vi "SPCReadFile.vi"(8 "Error In":errorcluster, 9 "Save data to ASCII":bool, 11 "SPC File":path) -> (0 "Error Out":errorcluster, 1 "Time Axis Multiplicator":dbl=0.01221522705078125, 2 "Events":u16[](array[numeric]) format="%04x", 3 "SumOfDecays":u32[](graph)=[0, 0, 0, 0, 0, 0, 0, 0, 0, 0, 0, 0, 0, 0, 0, 0, 0, 0, 0, 0, 0, 0, 0, 0, 0, 0, 0, 0, 0, 0, 0, 0, 0, 0, 0, 0, 0, 0, 0, 0, 0, 0, 0, 0, 0, 0, 0, 0, 0, 0, 0, 0, 0, 0, 0, 0, 0, 0, 0, 0, 0, 0, 0, 0, 0, 0, 0, 0, 0, 0, 0, 0, 0, 0, 0, 0, 0, 0, 0, 0, 0, 0, 0, 0, 0, 0, 0, 0, 0, 0, 0, 0, 0, 0, 0, 0, 0, 0, 0, 0, 0, 0, 0, 0, 0, 0, 0, 0, 0, 0, 0, 0, 0, 0, 0, 0, 0, 0, 0, 0, 0, 0, 0, 0, 0, 0, 0, 0, 0, 0, 0, 0, 0, 0, 0, 0, 0, 0, 0, 0, 0, 0, 0, 0, 0, 0, 0, 0, 0, 0, 0, 0, 0, 0, 0, 0, 0, 0, 0, 0, 0, 0, 0, 0, 0, 0, 0, 0, 0, 0, 0, 0, 0, 0, 0, 0, 0, 0, 0, 0, 0, 0, 0, 0, 0, 0, 0, 0, 0, 0, 0, 0, 0, 0, 0, 0, 0, 0, 0, 0, 0, 0, 0, 0, 0, 0, 0, 0, 0, 0, 0, 0, 0, 0, 0, 0, 0, 0, 0, 0, 0, 0, 0, 0, 0, 0, 0, 0, 0, 0, 0, 0, 0, 0, 0, 0, 0, 0, 0, 0, 0, 0, 0, 0, 0, 0, 0, 0, 0, 0, 0, 0, 0, 0, 0, 0, 0, 0, 0, 0, 0, 0, 0, 0, 0, 0, 0, 0, 0, 0, 0, 0, 0, 0, 0, 0, 0, 0, 0, 0, 0, 0, 0, 0, 0, 0, 0, 0, 0, 0, 0, 0, 0, 0, 0, 0, 0, 0, 0, 0, 0, 0, 0, 0, 0, 0, 0, 0, 0, 0, 0, 0, 0, 0, 0, 0, 0, 0, 0, 0, 0, 0, 0, 0, 0, 0, 0, 0, 0, 0, 0, 0, 0, 0, 0, 0, 0, 0, 0, 0, 0, 0, 0, 0, 0, 0, 0, 0, 0, 0, 0, 0, 0, 0, 0, 0, 0, 0, 0, 0, 0, 0, 0, 0, 0, 0, 0, 0, 0, 0, 0, 0, 0, 0, 0, 0, 0, 0, 0, 0, 0, 0, 0, 0, 0, 0, 0, 0, 0, 0, 0, 0, 0, 0, 0, 0, 0, 0, 0, 0, 0, 0, 0, 0, 0, 0, 0, 0, 0, 0, 0, 0, 0, 0, 0, 0, 0, 0, 0, 0, 0, 0, 0, 0, 0, 0, 0, 0, 0, 0, 0, 0, 0, 0, 0, 0, 0, 0, 0, 0, 0, 0, 0, 0, 0, 0, 0, 0, 0, 0, 0, 0, 0, 0, 0, 0, 0, 0, 0, 0, 0, 0, 0, 0, 0, 0, 0, 0, 0, 0, 0, 0, 0, 0, 0, 0, 0, 0, 0, 0, 0, 0, 0, 0, 0, 0, 0, 0, 0, 0, 0, 0, 0, 0, 0, 0, 0, 0, 0, 0, 0, 0, 0, 0, 0, 0, 0, 0, 0, 0, 0, 0, 0, 0, 0, 0, 0, 0, 0, 0, 0, 0, 0, 0, 0, 0, 0, 0, 0, 0, 0, 0, 0, 0, 0, 0, 0, 0, 0, 0, 0, 0, 0, 0, 0, 0, 0, 0, 0, 0, 0, 0, 0, 0, 0, 0, 0, 0, 0, 0, 0, 0, 0, 0, 0, 0, 0, 0, 0, 0, 0, 0, 0, 0, 0, 0, 0, 0, 0, 0, 0, 0, 0, 0, 0, 0, 0, 0, 0, 0, 0, 0, 0, 0, 0, 0, 0, 0, 0, 0, 0, 0, 0, 0, 0, 0, 0, 0, 0, 0, 0, 0, 0, 0, 0, 0, 0, 0, 0, 0, 0, 0, 0, 0, 0, 0, 0, 0, 0, 0, 0, 0, 0, 0, 0, 0, 0, 0, 0, 0, 0, 0, 0, 0, 0, 0, 0, 0, 0, 0, 0, 0, 0, 0, 0, 0, 0, 0, 0, 0, 0, 0, 0, 0, 0, 0, 0, 0, 0, 0, 0, 0, 0, 0, 0, 0, 0, 0, 0, 0, 0, 0, 0, 0, 0, 0, 0, 0, 0, 0, 0, 0, 0, 0, 0, 0, 0, 0, 0, 0, 0, 0, 0, 0, 0, 0, 0, 0, 0, 0, 0, 0, 0, 0, 0, 0, 0, 0, 0, 0, 0, 0, 0, 0, 0, 0, 0, 0, 0, 0, 0, 0, 0, 0, 0, 0, 0, 0, 0, 0, 0, 0, 0, 0, 0, 0, 0, 0, 0, 0, 0, 0, 0, 0, 0, 0, 0, 0, 0, 0, 0, 0, 0, 0, 0, 0, 0, 0, 0, 0, 0, 0, 0, 0, 0, 0, 0, 0, 0, 0, 0, 0, 0, 0, 0, 0, 0, 0, 0, 0, 0, 0, 0, 0, 0, 0, 0, 0, 0, 0, 0, 0, 0, 0, 0, 0, 0, 0, 0, 0, 0, 0, 0, 0, 0, 0, 0, 0, 0, 0, 0, 0, 0, 0, 0, 0, 0, 0, 0, 0, 0, 0, 0, 0, 0, 0, 0, 0, 0, 0, 0, 0, 0, 0, 0, 0, 0, 0, 0, 0, 0, 0, 0, 0, 0, 0, 0, 0, 0, 0, 0, 0, 0, 0, 0, 0, 0, 0, 0, 0, 0, 0, 0, 0, 0, 0, 0, 0, 0, 0, 0, 0, 0, 0, 0, 0, 0, 0, 0, 0, 0, 0, 0, 0, 0, 0, 0, 0, 0, 0, 0, 0, 0, 0, 0, 0, 0, 0, 0, 0, 0, 0, 0, 0, 0, 0, 0, 0, 0, 0, 0, 0, 0, 0, 0, 0, 0, 0, 0, 0, 0, 0, 0, 0, 0, 0, 0, 0, 0, 0, 0, 0, 0, 0, 0, 0, 0, 0, 0, 0, 0, 0, 0, 0, 0, 0, 0, 0, 0, 0, 0, 0, 0, 0, 0, 0, 0, 0, 0, 0, 0, 0, 0, 0, 0, 0, 0, 0, 0, 0, 0, 0, 0, 0, 0, 0, 0, 0, 0, 0, 0, 0, 0, 0, 0, 0, 0, 0, 0, 0, 0, 0, 0, 0, 0, 0, 0, 0, 0, 0, 0, 0, 0, 0, 0, 0, 0, 0, 0, 0, 0, 0, 0, 0, 0, 0, 0, 0, 0, 0, 0, 0, 0, 0, 0, 0, 0, 0, 0, 0, 0, 0, 0, 0, 0, 0, 0, 0, 0, 0, 0, 0, 0, 0, 0, 0, 0, 0, 0, 0, 0, 0, 0, 0, 0, 0, 0, 0, 0, 0, 0, 0, 0, 0, 0, 0, 0, 0, 0, 0, 0, 0, 0, 0, 0, 0, 0, 0, 0, 0, 0, 0, 0, 0, 0, 0, 0, 0, 0, 0, 0, 0, 0, 0, 0, 0, 0, 0, 0, 0, 0, 0, 0, 0, 0, 0, 0, 0, 0, 0, 0, 0, 0, 0, 0, 0, 0, 0, 0, 0, 0, 0, 0, 0, 0, 0, 0, 0, 0, 0, 0, 0, 0, 0, 0, 0, 0, 0, 0, 0, 0, 0, 0, 0, 0, 0, 0, 0, 0, 0, 0, 0, 0, 0, 0, 0, 0, 0, 0, 0, 0, 0, 0, 0, 0, 0, 0, 0, 0, 0, 0, 0, 0, 0, 0, 0, 0, 0, 0, 0, 0, 0, 0, 0, 0, 0, 0, 0, 0, 0, 0, 0, 0, 0, 0, 0, 0, 0, 0, 0, 0, 0, 0, 0, 0, 0, 0, 0, 0, 0, 0, 0, 0, 0, 0, 0, 0, 0, 0, 0, 0, 0, 0, 0, 0, 0, 0, 0, 0, 0, 0, 0, 0, 0, 0, 0, 0, 0, 0, 0, 0, 0, 0, 0, 0, 0, 0, 0, 0, 0, 0, 0, 0, 0, 0, 0, 0, 0, 0, 0, 0, 0, 0, 0, 0, 0, 0, 0, 0, 0, 0, 0, 0, 0, 0, 0, 0, 0, 0, 0, 0, 0, 0, 0, 0, 0, 0, 0, 0, 0, 0, 0, 0, 0, 0, 0, 0, 0, 0, 0, 0, 0, 0, 0, 0, 0, 0, 0, 0, 0, 0, 0, 0, 0, 0, 0, 0, 0, 0, 0, 0, 0, 0, 0, 0, 0, 0, 0, 0, 0, 0, 0, 0, 0, 0, 0, 0, 0, 0, 0, 0, 0, 0, 0, 0, 0, 0, 0, 0, 0, 0, 0, 0, 0, 0, 0, 0, 0, 0, 0, 0, 0, 0, 0, 0, 0, 0, 0, 0, 0, 0, 0, 0, 0, 0, 0, 0, 0, 0, 0, 0, 0, 0, 0, 0, 0, 0, 0, 0, 0, 0, 0, 0, 0, 0, 0, 0, 0, 0, 0, 0, 0, 0, 0, 0, 0, 0, 0, 0, 0, 0, 0, 0, 0, 0, 0, 0, 0, 0, 0, 0, 0, 0, 0, 0, 0, 0, 0, 0, 0, 0, 0, 0, 0, 0, 0, 0, 0, 0, 0, 0, 0, 0, 0, 0, 0, 0, 0, 0, 0, 0, 0, 0, 0, 0, 0, 0, 0, 0, 0, 0, 0, 0, 0, 0, 0, 0, 0, 0, 0, 0, 0, 0, 0, 0, 0, 0, 0, 0, 0, 0, 0, 0, 0, 0, 0, 0, 0, 0, 0, 0, 0, 0, 0, 0, 0, 0, 0, 0, 0, 0, 0, 0, 0, 0, 0, 0, 0, 0, 0, 0, 0, 0, 0, 0, 0, 0, 0, 0, 0, 0, 0, 0, 0, 0, 0, 0, 0, 0, 0, 0, 0, 0, 0, 0, 0, 0, 0, 0, 0, 0, 0, 0, 0, 0, 0, 0, 0, 0, 0, 0, 0, 0, 0, 0, 0, 0, 0, 0, 0, 0, 0, 0, 0, 0, 0, 0, 0, 0, 0, 0, 0, 0, 0, 0, 0, 0, 0, 0, 0, 0, 0, 0, 0, 0, 0, 0, 0, 0, 0, 0, 0, 0, 0, 0, 0, 0, 0, 0, 0, 0, 0, 0, 0, 0, 0, 0, 0, 0, 0, 0, 0, 0, 0, 0, 0, 0, 0, 0, 0, 0, 0, 0, 0, 0, 0, 0, 0, 0, 0, 0, 0, 0, 0, 0, 0, 0, 0, 0, 0, 0, 0, 0, 0, 0, 0, 0, 0, 0, 0, 0, 0, 0, 0, 0, 0, 0, 0, 0, 0, 0, 0, 0, 0, 0, 0, 0, 0, 0, 0, 0, 0, 0, 0, 0, 0, 0, 0, 0, 0, 0, 0, 0, 0, 0, 0, 0, 0, 0, 0, 0, 0, 0, 0, 0, 0, 0, 0, 0, 0, 0, 0, 0, 0, 0, 0, 0, 0, 0, 0, 0, 0, 0, 0, 0, 0, 0, 0, 0, 0, 0, 0, 0, 0, 0, 0, 0, 0, 0, 0, 0, 0, 0, 0, 0, 0, 0, 0, 0, 0, 0, 0, 0, 0, 0, 0, 0, 0, 0, 0, 0, 0, 0, 0, 0, 0, 0, 0, 0, 0, 0, 0, 0, 0, 0, 0, 0, 0, 0, 0, 0, 0, 0, 0, 0, 0, 0, 0, 0, 0, 0, 0, 0, 0, 0, 0, 0, 0, 0, 0, 0, 0, 0, 0, 0, 0, 0, 0, 0, 0, 0, 0, 0, 0, 0, 0, 0, 0, 0, 0, 0, 0, 0, 0, 0, 0, 0, 0, 0, 0, 0, 0, 0, 0, 0, 0, 0, 0, 0, 0, 0, 0, 0, 0, 0, 0, 0, 0, 0, 0, 0, 0, 0, 0, 0, 0, 0, 0, 0, 0, 0, 0, 0, 0, 0, 0, 0, 0, 0, 0, 0, 0, 0, 0, 0, 0, 0, 0, 0, 0, 0, 0, 0, 0, 0, 0, 0, 0, 0, 0, 0, 0, 0, 0, 0, 0, 0, 0, 0, 0, 0, 0, 0, 0, 0, 0, 0, 0, 0, 0, 0, 0, 0, 0, 0, 0, 0, 0, 0, 0, 0, 0, 0, 0, 0, 0, 0, 0, 0, 0, 0, 0, 0, 0, 0, 0, 0, 0, 0, 0, 0, 0, 0, 0, 0, 0, 0, 0, 0, 0, 0, 0, 0, 0, 0, 0, 0, 0, 0, 0, 0, 0, 0, 0, 0, 0, 0, 0, 0, 0, 0, 0, 0, 0, 0, 0, 0, 0, 0, 0, 0, 0, 0, 0, 0, 0, 0, 0, 0, 0, 0, 0, 0, 0, 0, 0, 0, 0, 0, 0, 0, 0, 0, 0, 0, 0, 0, 0, 0, 0, 0, 0, 0, 0, 0, 0, 0, 0, 0, 0, 0, 0, 0, 0, 0, 0, 0, 0, 0, 0, 0, 0, 0, 0, 0, 0, 0, 0, 0, 0, 0, 0, 0, 0, 0, 0, 0, 0, 0, 0, 0, 0, 0, 0, 0, 0, 0, 0, 0, 0, 0, 0, 0, 0, 0, 0, 0, 0, 0, 0, 0, 0, 0, 0, 0, 0, 0, 0, 0, 0, 0, 0, 0, 0, 0, 0, 0, 0, 0, 0, 0, 0, 0, 0, 0, 0, 0, 0, 0, 0, 0, 0, 0, 0, 0, 0, 0, 0, 0, 0, 0, 0, 0, 0, 0, 0, 0, 0, 0, 0, 0, 0, 0, 0, 0, 0, 0, 0, 0, 0, 0, 0, 0, 0, 0, 0, 0, 0, 0, 0, 0, 0, 0, 0, 0, 0, 0, 0, 0, 0, 0, 0, 0, 0, 0, 0, 0, 0, 0, 0, 0, 0, 0, 0, 0, 0, 0, 0, 0, 0, 0, 0, 0, 0, 0, 0, 0, 0, 0, 0, 0, 0, 0, 0, 0, 0, 0, 0, 0, 0, 0, 0, 0, 0, 0, 0, 0, 0, 0, 0, 0, 0, 0, 0, 0, 0, 0, 0, 0, 0, 0, 0, 0, 0, 0, 0, 0, 0, 0, 0, 0, 0, 0, 0, 0, 0, 0, 0, 0, 0, 0, 0, 0, 0, 0, 0, 0, 0, 0, 0, 0, 0, 0, 0, 0, 0, 0, 0, 0, 0, 0, 0, 0, 0, 0, 0, 0, 0, 0, 0, 0, 0, 0, 0, 0, 0, 0, 0, 0, 0, 0, 0, 0, 0, 0, 0, 0, 0, 0, 0, 0, 0, 0, 0, 0, 0, 0, 0, 0, 0, 0, 0, 0, 0, 0, 0, 0, 0, 0, 0, 0, 0, 0, 0, 0, 0, 0, 0, 0, 0, 0, 0, 0, 0, 0, 0, 0, 0, 0, 0, 0, 0, 0, 0, 0, 0, 0, 0, 0, 0, 0, 0, 0, 0, 0, 0, 0, 0, 0, 0, 0, 0, 0, 0, 0, 0, 0, 0, 0, 0, 0, 0, 0, 0, 0, 0, 0, 0, 0, 0, 0, 0, 0, 0, 0, 0, 0, 0, 0, 0, 0, 0, 0, 0, 0, 0, 0, 0, 0, 0, 0, 0, 0, 0, 0, 0, 0, 0, 0, 0, 0, 0, 0, 0, 0, 0, 0, 0, 0, 0, 0, 0, 0, 0, 0, 0, 0, 0, 0, 0, 0, 0, 0, 0, 0, 0, 0, 0, 0, 0, 0, 0, 0, 0, 0, 0, 0, 0, 0, 0, 0, 0, 0, 0, 0, 0, 0, 0, 0, 0, 0, 0, 0, 0, 0, 0, 0, 0, 0, 0, 0, 0, 0, 0, 0, 0, 0, 0, 0, 0, 0, 0, 0, 0, 0, 0, 0, 0, 0, 0, 0, 0, 0, 0, 0, 0, 0, 0, 0, 0, 0, 0, 0, 0, 0, 0, 0, 0, 0, 0, 0, 0, 0, 0, 0, 0, 0, 0, 0, 0, 0, 0, 0, 0, 0, 0, 0, 0, 0, 0, 0, 0, 0, 0, 0, 0, 0, 0, 0, 0, 0, 0, 0, 0, 0, 0, 0, 0, 0, 0, 0, 0, 0, 0, 0, 0, 0, 0, 0, 0, 0, 0, 0, 0, 0, 0, 0, 0, 0, 0, 0, 0, 0, 0, 0, 0, 0, 0, 0, 0, 0, 0, 0, 0, 0, 0, 0, 0, 0, 0, 0, 0, 0, 0, 0, 0, 0, 0, 0, 0, 0, 0, 0, 0, 0, 0, 0, 0, 0, 0, 0, 0, 0, 0, 0, 0, 0, 0, 0, 0, 0, 0, 0, 0, 0, 0, 1, 1, 0, 4, 14, 38, 73, 95, 122, 99, 134, 110, 126, 111, 113, 126, 115, 121, 109, 122, 113, 114, 107, 104, 107, 132, 100, 108, 122, 112, 119, 107, 110, 110, 118, 112, 92, 122, 88, 118, 121, 113, 109, 116, 112, 120, 109, 97, 94, 101, 103, 105, 117, 117, 100, 103, 105, 105, 100, 108, 117, 122, 124, 112, 87, 106, 126, 133, 114, 98, 108, 94, 98, 102, 85, 99, 120, 100, 80, 90, 119, 104, 93, 111, 117, 109, 96, 98, 96, 92, 105, 105, 123, 77, 96, 110, 114, 112, 92, 96, 105, 80, 92, 100, 99, 94, 83, 101, 98, 94, 96, 105, 113, 96, 93, 104, 104, 103, 77, 92, 93, 108, 93, 83, 98, 84, 110, 96, 91, 104, 72, 86, 79, 96, 90, 75, 90, 101, 102, 89, 92, 80, 105, 92, 104, 103, 77, 98, 81, 97, 96, 97, 107, 92, 82, 99, 88, 74, 78, 91, 85, 83, 95, 89, 72, 83, 108, 66, 77, 98, 85, 86, 77, 99, 89, 105, 126, 187, 349, 597, 975, 1527, 2330, 2969, 3879, 4539, 5078, 5604, 6137, 6593, 6955, 7051, 7400, 7634, 7591, 7692, 7829, 7947, 7715, 7869, 7800, 7720, 7689, 7584, 7563, 7526, 7329, 7329, 7218, 7194, 7152, 7039, 6914, 6778, 6874, 6667, 6393, 6476, 6322, 6350, 6081, 5926, 5805, 5859, 5729, 5629, 5567, 5332, 5420, 5262, 5094, 5102, 4896, 4954, 4887, 4802, 4602, 4611, 4606, 4518, 4273, 4291, 4253, 4182, 4187, 4141, 4033, 3926, 4019, 3933, 3905, 3889, 3746, 3637, 3618, 3581, 3610, 3562, 3485, 3445, 3529, 3453, 3306, 3258, 3248, 3195, 3087, 3145, 3066, 3049, 2997, 2980, 3002, 2907, 2886, 2905, 2833, 2676, 2766, 2723, 2635, 2718, 2619, 2556, 2518, 2584, 2525, 2519, 2578, 2409, 2465, 2473, 2396, 2457, 2379, 2350, 2402, 2311, 2353, 2399, 2259, 2181, 2159, 2300, 2133, 2170, 2173, 2080, 2064, 2210, 2052, 1969, 2048, 2040, 2017, 1909, 2036, 2036, 2046, 1892, 1929, 1853, 1943, 1859, 1893, 1875, 1860, 1760, 1837, 1739, 1768, 1731, 1737, 1696, 1641, 1691, 1699, 1704, 1650, 1605, 1646, 1596, 1539, 1559, 1605, 1626, 1527, 1510, 1548, 1535, 1511, 1493, 1479, 1507, 1457, 1409, 1506, 1476, 1440, 1374, 1453, 1411, 1383, 1432, 1386, 1452, 1346, 1351, 1312, 1363, 1357, 1305, 1312, 1278, 1295, 1260, 1257, 1269, 1206, 1268, 1268, 1281, 1231, 1215, 1220, 1216, 1270, 1245, 1177, 1128, 1138, 1152, 1121, 1118, 1116, 1110, 1128, 1072, 1120, 1060, 1135, 1055, 1114, 1056, 1019, 1061, 1132, 1051, 1000, 1041, 1057, 1018, 977, 975, 994, 1010, 949, 937, 1025, 990, 965, 1005, 979, 966, 904, 905, 948, 904, 877, 908, 882, 904, 890, 950, 944, 868, 859, 895, 836, 842, 820, 870, 817, 821, 789, 897, 795, 784, 886, 839, 756, 769, 813, 824, 829, 781, 794, 790, 827, 823, 788, 826, 742, 824, 760, 749, 749, 767, 798, 757, 735, 748, 670, 730, 711, 744, 729, 713, 646, 679, 722, 713, 679, 702, 679, 705, 688, 670, 652, 677, 700, 672, 681, 582, 724, 682, 669, 675, 677, 647, 632, 611, 638, 671, 622, 609, 629, 585, 623, 560, 560, 613, 608, 635, 619, 606, 609, 563, 613, 592, 553, 581, 536, 555, 582, 539, 556, 593, 536, 556, 526, 548, 537, 505, 531, 539, 515, 521, 529, 488, 551, 550, 529, 529, 531, 489, 500, 497, 509, 483, 514, 466, 494, 495, 508, 515, 497, 518, 490, 487, 475, 511, 542, 503, 476, 483, 449, 502, 482, 472, 455, 464, 524, 463, 438, 461, 478, 475, 488, 445, 453, 461, 448, 422, 442, 425, 423, 482, 435, 427, 408, 441, 451, 442, 471, 441, 414, 443, 442, 402, 404, 405, 422, 424, 405, 386, 417, 400, 398, 400, 376, 445, 401, 404, 392, 397, 357, 353, 358, 386, 402, 399, 402, 376, 403, 377, 385, 386, 323, 342, 374, 361, 356, 363, 383, 382, 371, 317, 362, 355, 353, 407, 380, 403, 350, 336, 340, 348, 337, 372, 330, 371, 333, 346, 346, 365, 297, 315, 313, 355, 332, 319, 325, 301, 305, 337, 330, 346, 346, 348, 306, 291, 304, 342, 334, 312, 287, 309, 315, 303, 314, 314, 308, 308, 276, 298, 338, 308, 312, 321, 311, 308, 280, 293, 309, 291, 307, 276, 301, 293, 299, 297, 254, 279, 299, 307, 243, 267, 276, 283, 260, 264, 294, 286, 294, 271, 280, 243, 305, 262, 272, 278, 281, 289, 269, 266, 265, 285, 258, 251, 274, 284, 248, 254, 258, 259, 287, 247, 283, 268, 240, 260, 268, 249, 240, 247, 293, 245, 285, 271, 237, 239, 260, 261, 236, 242, 240, 202, 253, 238, 221, 207, 266, 228, 226, 229, 241, 215, 237, 224, 254, 226, 200, 191, 222, 212, 194, 246, 210, 230, 259, 215, 212, 201, 244, 194, 205, 226, 200, 195, 211, 239, 223, 210, 199, 204, 223, 209, 215, 214, 233, 227, 230, 220, 211, 225, 188, 216, 183, 223, 202, 206, 201, 200, 208, 185, 218, 206, 207, 219, 210, 195, 195, 183, 205, 182, 181, 183, 210, 212, 190, 181, 199, 206, 204, 178, 181, 191, 200, 193, 191, 190, 196, 196, 202, 169, 196, 183, 207, 180, 190, 177, 168, 187, 203, 165, 174, 199, 179, 194, 168, 159, 164, 181, 191, 162, 170, 166, 172, 168, 205, 174, 189, 159, 153, 185, 176, 186, 170, 179, 173, 178, 183, 162, 159, 171, 182, 176, 147, 157, 161, 151, 166, 173, 150, 171, 152, 159, 178, 176, 153, 146, 173, 156, 158, 157, 162, 132, 163, 140, 165, 164, 182, 144, 166, 151, 163, 156, 154, 160, 134, 141, 148, 148, 143, 145, 138, 144, 180, 138, 137, 152, 151, 152, 154, 150, 174, 143, 132, 153, 124, 150, 157, 135, 150, 154, 130, 160, 145, 140, 127, 147, 134, 143, 154, 125, 133, 135, 145, 137, 149, 134, 160, 135, 143, 131, 129, 133, 142, 149, 154, 154, 133, 106, 136, 120, 156, 156, 136, 130, 142, 154, 137, 147, 140, 150, 133, 154, 126, 139, 131, 126, 142, 122, 129, 127, 125, 137, 134, 112, 126, 133, 116, 118, 131, 128, 128, 137, 125, 116, 150, 125, 153, 129, 138, 126, 146, 143, 120, 175, 163, 212, 235, 248, 193, 105, 28, 10, 2, 1, 1, 0, 1, 0, 0, 0, 0, 0, 0, 0, 0, 0, 0, 0, 0, 1, 1, 0, 0, 0, 0, 0, 0, 0, 0, 0, 0, 0, 0, 0, 0, 0, 0, 0, 0, 0, 0, 0, 0, 0, 0, 0, 0, 0, 0, 0, 0, 0, 0, 0, 0, 0, 0, 0, 0, 0, 0, 0, 0, 0, 0, 0, 0, 0, 0, 0, 0, 0, 0, 0, 0, 0, 0, 0, 0, 0, 0, 0, 0, 0, 0, 0, 0, 0, 0, 0, 0, 0, 0, 0, 0, 0, 0, 0, 0, 0, 0, 0, 0, 0, 0, 0, 0, 0, 0, 0, 0, 0, 0, 0, 0, 0, 0, 0, 0, 0, 0, 0, 0, 0, 0, 0, 0, 0, 0, 0, 0, 0, 0, 0, 0, 0, 0, 0, 0, 0, 0, 0, 0, 0, 0, 0, 0, 0, 0, 0, 0, 0, 0, 0, 0, 0, 0, 0, 0, 0, 0, 0, 0, 0, 0, 0, 0, 0, 0, 0, 0, 0, 0, 0, 0, 0, 0, 0, 0, 0, 0, 0, 0, 0, 0, 0, 0, 0, 0, 0, 0, 0, 0, 0, 0, 0, 0, 0, 0, 0, 0, 0, 0, 0, 0, 0, 0, 0, 0, 0, 0, 0, 0, 0, 0, 0, 0, 0, 0, 0, 0, 0, 0, 0, 0, 0, 0, 0, 0, 0, 0, 0, 0, 0, 0, 0, 0, 0, 0, 0, 0, 0, 0, 0, 0, 0, 0, 0, 0, 0, 0, 0, 0, 0, 0, 0, 0, 0, 0, 0, 0, 0, 0, 0, 0, 0, 0, 0, 0, 0, 0, 0, 0, 0, 0, 0, 0, 0, 0, 0, 0, 0, 0, 0, 0, 0, 0, 0, 0, 0, 0, 0, 0, 0, 0, 0, 0, 0, 0, 0, 0, 0, 0, 0, 0, 0, 0, 0, 0, 0, 0, 0, 0, 0, 0, 0, 0, 0, 0, 0, 0, 0, 0, 0, 0, 0, 0, 0, 0, 0, 0, 0, 0, 0, 0, 0, 0, 0, 0, 0, 0, 0, 0, 0, 0, 0, 0, 0, 0, 0, 0, 0, 0, 0, 0, 0, 0, 0, 0, 0, 0, 0, 0, 0, 0, 0, 0, 0, 0, 0, 0, 0, 0, 0, 0, 0, 0, 0, 0, 0, 0, 0, 0, 0, 0, 0, 0, 0, 0, 0, 0, 0, 0, 0, 0, 0, 0, 0, 0, 0, 0, 0, 0, 0, 0, 0, 0, 0, 0, 0, 0, 0, 0, 0, 0, 0, 0, 0, 0, 0, 0, 0, 0, 0, 0, 0, 0, 0, 0, 0, 0, 0, 0, 0, 0, 0, 0, 0, 0, 0, 0, 0, 0, 0, 0, 0, 0, 0, 0, 0, 0, 0, 0, 0, 0, 0, 0, 0, 0, 0, 0, 0, 0, 0], 4 "PhotonCount":u64, 5 "Macro Time Clk":dbl=0.012215228751301765, 6 "File with Marker":bool, 7 "NoOfRoutingChannels":u16)   [LabVIEW 2023]
doc: "This VI reads a SPC-/SET-file pair from disc. The header and event data are interpreted and displayed. The graph's Time Axis is scaled using the information stored in the SET-file.\n<b>Note:</b> Events are always 2 word wide, and received in reversed byte and word order.\nOptional the Events can be written to a *.csv file.\nFor a description of the *.set file format see: SPC_data_file_structure.h\nUse this VI to display data stored previously in a SPC-/SET-file pair or to create your own analysis on this data. \n\ninfo@becker-hickl.com"
uses:
  <vilib>/Utility/file.llb/Write Delimited Spreadsheet (I64).vi
panel:
  out "EventHeader":u32 format="%08x"
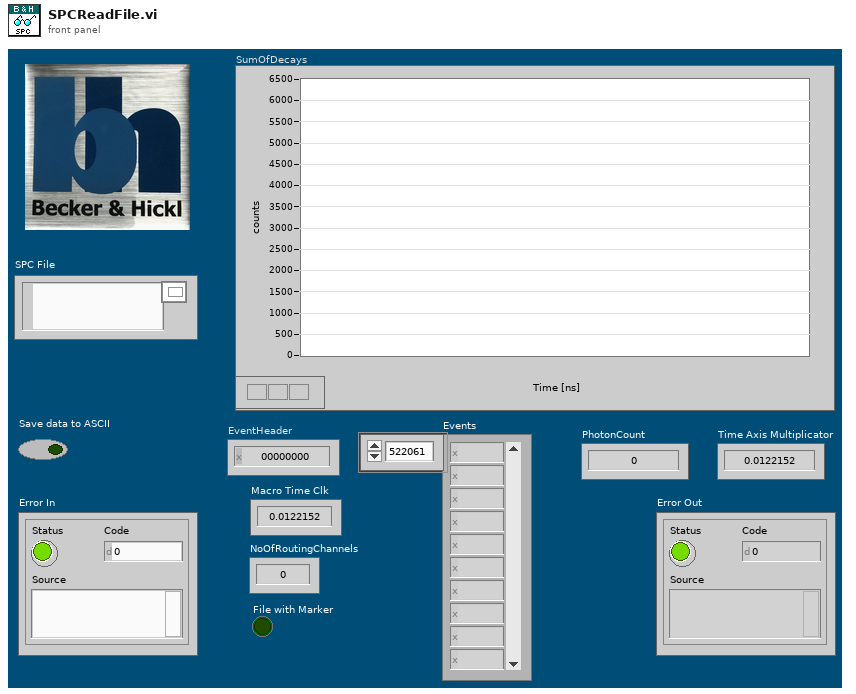
[diagram p1: front panel]
types:
  T1 = enum16{"open", "replace", "create", "open or create", "replace or create", "replace or create with confirmation"}
  T2 = enum16{"big-endian, network order", "native, host order", "little-endian"}
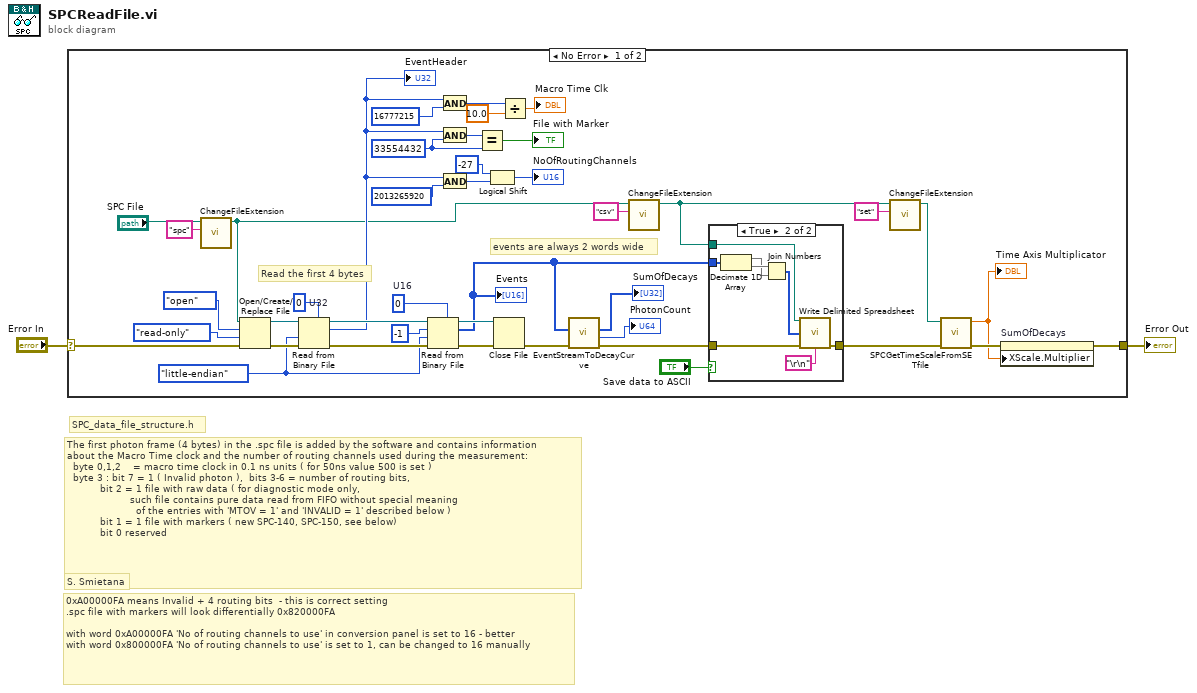
[diagram p0: block diagram]
diagram:
  # "S. Smietana"
  # "0xA00000FA means Invalid + 4 routing bits  - this is correct setting\n.spc file with markers will look differentially 0x820000FA\n\nwith word 0xA00000FA 'No of routing channels to use' in conversion panel is set to 16 - better\nwith word 0x800000FA 'No of routing channels to use' is set to 1, can be changed to 16 manually"
  # "SPC_data_file_structure.h"
  # "The first photon frame (4 bytes) in the .spc file is added by the software and contains information \nabout the Macro Time clock and the number of routing channels used during the measurement:\n  byte 0,1,2    = macro time clock in 0.1 ns units ( for 50ns value 500 is set )\n  byte 3 : bit 7 = 1 ( Invalid photon ),  bits 3-6 = number of routing bits, \n           bit 2 = 1 file with raw data ( for diagnostic mode only, \n                     such file contains pure data read from FIFO without special meaning \n                       of the entries with 'MTOV = 1' and 'INVALID = 1' described below )\n           bit 1 = 1 file with markers ( new SPC-140, SPC-150, see below)\n           bit 0 reserved"
  n1 = case shown="No Error" "Error In" {
    selector: "Error In" -> [w37 w54]
    tunnel: [w11 w54] -> w2
    frame No Error {
      w16 = u32 33554432
      w32 = u32 0  # U32
      w35 = u16 0  # U16
      w31 = T2."little-endian" ("byte order (0:big-endian, network order)")
      # "events are always 2 words wide"
      # "Read the first 4 bytes"
      n2 = call "ChangeFileExtension.vi"("NewExtension"="spc", "OldPath"="SPC File") -> ("NewPath"=w4:path)  [unwired: 8 in, 1 out]
      n3 = Open/Create/Replace File(file path (use dialog)=w4, error in=w37, operation (0:open)=T1."open", access (0:read/write)=enum16{"read/write", "read-only", "write-only"}."read-only") -> (refnum out=w38:refnum<file>, error out=w42:errorcluster)  [unwired: 2 in, 1 out]
      n4 = Read from Binary File(5:w32, 8:w42, 9:w31, 11:w38) -> (0:w33:errorcluster, 2:w15:u32, 3:w34:refnum<file>)  [unwired: 2 in, 1 out]
      "EventHeader" <- w15
      n5 = Read from Binary File(5:w35, 8:w33, 9:w31, 10:-1 ("count (1)"), 11:w34) -> (0:w29:errorcluster, 2:w27:u16[], 3:w30:refnum<file>)  [unwired: 1 in, 1 out]
      "Events" <- w27
      n6 = And(x=w15, y=u32 16777215) -> (x .and. y?=w24:u32)
      n7 = And(x=w15, y=w16) -> (x .and. y?=w17:u32)
      n8 = And(x=w15, y=u32 2013265920) -> (x .and. y?=w20:u32)
      n9 = Equal?(x=w17, y=w16) -> (x = y?=→"File with Marker":bool)
      n10 = Logical Shift(y=i16 -27, x=w20) -> (x << y=→"NoOfRoutingChannels":u32)
      n11 = Close File(refnum=w30, error in=w29) -> (error out=w14:errorcluster)  [unwired: 1 out]
      n12 = Divide(x=w24, y=10.0) -> (x/y=→"Macro Time Clk":dbl)
      n13 = call "EventStreamToDecayCurve.vi"("Error In"=w14, "EventData"=w27) -> ("Error Out"=w26:errorcluster, "PhotonCount"=→"PhotonCount":u64, "DecaySum"=→"SumOfDecays":u32[])  [unwired: 4 in, 3 out]
      n14 = call "ChangeFileExtension.vi"("NewExtension"="csv", "OldPath"=w4) -> ("NewPath"=w3:path)  [unwired: 8 in, 1 out]
      n15 = case shown="True" "Save data to ASCII" {
        tunnel: w26 -> [w45 w53]
        tunnel: [w45 w52] -> w13
        tunnel: w27 -> [_ w49]
        tunnel: w3 -> [_ w47]
        frame False {
        }
        frame True {
          n16 = Decimate 1D Array(w49) -> (w50:u16[], w51:u16[])
          n17 = Join Numbers(hi=w51, lo=w50) -> ((hi.lo)=w48:u32[])
          n18 = call-poly <vilib>:"Write Delimited Spreadsheet.vi"("file path (dialog if empty)"=w47, "1D data"=w48, "error in (no error)"=w53, "delimiter (\\t)"="\r\n") -> ("error out"=w52:errorcluster)  [unwired: 10 in, 1 out]
        }
      }
      n19 = call "ChangeFileExtension.vi"("NewExtension"="set", "OldPath"=w3) -> ("NewPath"=w6:path)  [unwired: 8 in, 1 out]
      n20 = call "SPCGetTimeScaleFromSETfile.vi"("error in"=w13, "setFile"=w6) -> ("error out"=w12:errorcluster, "TimeAxisMultiplicator"=w10:dbl)  [unwired: 2 in, 6 out]
      "Time Axis Multiplicator" <- w10
      n21 = property on="SumOfDecays" class="WFGraph (strict)"(error in=w12, "XScale.Multiplier"=w10) -> (error out=w11:errorcluster)  [unwired: 1 in, 1 out]
    }
    frame Error {
    }
  }
  "Error Out" <- w2
